vi "Experiment_CAVITY.vi"() -> ()   [LabVIEW 2009]
uses:
  <vilib>/imath/engines/lvmath2/RunTimeEngine/ErrorHandling/NIMS_Finalize Error.vi
  <vilib>/imath/engines/lvmath2/RunTimeEngine/Parser/MC_Version.vi
  <vilib>/imath/engines/lvmath2/RunTimeEngine/Managers/WorkSpace/UID Generator.vi
  <vilib>/imath/engines/lvmath2/RunTimeEngine/NodeEndStatement/NIMS_NodeEndStatement_Output.vi
  <instcachedir>/0/NIMS_NodeEndStatement_Output_B70DDD75627E4997AAE11E9955EDAA25.lvgen/NIMS_NodeEndStatement_Output_B70DDD75627E4997AAE11E9955EDAA25_001.vi
  <vilib>/imath/engines/lvmath2/RunTimeEngine/Managers/SymbolTable/Clear UID.vi
  <vilib>/imath/engines/lvmath2/RunTimeEngine/LocalVariableDefStatement/MC_LocalVariableDefStatement_Display.vi
  <vilib>/imath/engines/lvmath2/RunTimeEngine/RunTimeType/NIMS_RunTimeType_From StrictType (excl LVString).vi
  <vilib>/imath/engines/lvmath2/RunTimeEngine/RangeToken/NIMS_Range.vi
  <instcachedir>/0/NIMS_Range_6D647EC16A744C98B5DE1D649A2D648D.lvgen/NIMS_Range_6D647EC16A744C98B5DE1D649A2D648D_001.vi
  <vilib>/imath/engines/lvmath/Functions/Error Handling/error.ctl
  <vilib>/imath/engines/lvmath/Functions/Error Handling/MergeErrorsWrapper.vi
  <vilib>/imath/engines/lvmath2/RunTimeEngine/VariableToken/NIMS_VariableToken_CondDefined.vi
  <instcachedir>/0/NIMS_VariableToken_CondDefined_5641E79000FB4D628475532441475385.lvgen/NIMS_VariableToken_CondDefined_5641E79000FB4D628475532441475385_002.vi
  <vilib>/imath/engines/lvmath/Functions/Error Handling/MC_Mask_Errors.vi
  <vilib>/imath/engines/lvmath2/RunTimeEngine/BuiltInFunctions/rem/NIMS_rem_no checks.vi
  <instcachedir>/0/NIMS_rem_no checks_4CC9B305AB7E42EF90AFC4973FB32F8D.lvgen/NIMS_rem_no checks_4CC9B305AB7E42EF90AFC4973FB32F8D_000.vi
  <vilib>/imath/engines/lvmath2/RunTimeEngine/BuiltInFunctions/uint32/NIMS_uint32(real).vi
  <instcachedir>/0/NIMS_uint32(real)_FDC83D68D45943DDB8F3F934FF8A712F.lvgen/NIMS_uint32(real)_FDC83D68D45943DDB8F3F934FF8A712F_000.vi
  <vilib>/imath/engines/lvmath2/RunTimeEngine/BuiltInFunctions/double/NIMS_double.vi
  <instcachedir>/0/NIMS_double_2CE444F3CE4146B199A482FE12545E45.lvgen/NIMS_double_2CE444F3CE4146B199A482FE12545E45_000.vi
  <vilib>/imath/engines/lvmath2/RunTimeEngine/BuiltInFunctions/length/NIMS_length(GV).vi
  <instcachedir>/0/NIMS_length(GV)_7D6E94E728E145E68721C53861296D96.lvgen/NIMS_length(GV)_7D6E94E728E145E68721C53861296D96_000.vi
  <instcachedir>/0/NIMS_Range_6D647EC16A744C98B5DE1D649A2D648D.lvgen/NIMS_Range_6D647EC16A744C98B5DE1D649A2D648D_000.vi
  <vilib>/imathl/engines/lvmath/Functions/Error Handling/Create Error.vi
  <vilib>/imath/engines/lvmath2/RunTimeEngine/ReplaceToken/NIMS_Replace - V(S)=S.vi
  <instcachedir>/0/NIMS_Replace - V(S)=S_670A9E0533664C1D848C8E58B3321B6A.lvgen/NIMS_Replace - V(S)=S_670A9E0533664C1D848C8E58B3321B6A_001.vi
  <vilib>/imath/engines/lvmath2/RunTimeEngine/ReplaceToken/NIMS_Replace - Size Check _(_)=S.vi
  <instcachedir>/0/NIMS_Replace - Size Check _(_)=S_8596181D73404097BAB9CBB006194BB0.lvgen/NIMS_Replace - Size Check _(_)=S_8596181D73404097BAB9CBB006194BB0_002.vi
  <vilib>/imath/engines/lvmath2/RunTimeEngine/ReplaceToken/NIMS_Replace - Check Linear.vi
  <instcachedir>/0/NIMS_Replace - Check Linear_9243CBB174894FF6977027453DA6955E.lvgen/NIMS_Replace - Check Linear_9243CBB174894FF6977027453DA6955E_002.vi
  <vilib>/imath/engines/lvmath2/RunTimeEngine/VariableToken/NIMS_VariableToken_CondDefinedDefinedByReplace.vi
  <instcachedir>/0/NIMS_VariableToken_CondDefinedDefinedByReplace_D162CFFC24174562A9FEA619A91E1A56.lvgen/NIMS_VariableToken_CondDefinedDefinedByReplace_D162CFFC24174562A9FEA619A91E1A56_002.vi
  <vilib>/imath/engines/lvmath2/RunTimeEngine/CommandStatement/MC_CommandStatement_break.vi
  <vilib>/imath/engines/lvmath2/RunTimeEngine/ArithmeticOperatorToken/NIMS_ArithmeticOperator_times.vi
  <instcachedir>/0/NIMS_ArithmeticOperator_times_3987BC660D7947CD8628C10658A43225.lvgen/NIMS_ArithmeticOperator_times_3987BC660D7947CD8628C10658A43225_001.vi
  <instcachedir>/0/NIMS_NodeEndStatement_Output_B70DDD75627E4997AAE11E9955EDAA25.lvgen/NIMS_NodeEndStatement_Output_B70DDD75627E4997AAE11E9955EDAA25_000.vi
  <instcachedir>/0/NIMS_ArithmeticOperator_times_3987BC660D7947CD8628C10658A43225.lvgen/NIMS_ArithmeticOperator_times_3987BC660D7947CD8628C10658A43225_000.vi
  <vilib>/imath/engines/lvmath2/RunTimeEngine/VariableToken/Read/NIMS_Get Elements - RV(_) - Check.vi
  <instcachedir>/0/NIMS_Get Elements - RV(_) - Check_60F12861D0564803969A5D0D0D1716CD.lvgen/NIMS_Get Elements - RV(_) - Check_60F12861D0564803969A5D0D0D1716CD_001.vi
  <instcachedir>/0/NIMS_VariableToken_CondDefined_5641E79000FB4D628475532441475385.lvgen/NIMS_VariableToken_CondDefined_5641E79000FB4D628475532441475385_001.vi
  <instcachedir>/0/NIMS_VariableToken_CondDefined_5641E79000FB4D628475532441475385.lvgen/NIMS_VariableToken_CondDefined_5641E79000FB4D628475532441475385_003.vi
  <vilib>/imath/engines/lvmath2/RunTimeEngine/ArithmeticOperatorToken/NIMS_ArithmeticOperator_power(S).vi
  <instcachedir>/0/NIMS_ArithmeticOperator_power(S)_A502679C095F4520BDC53E297C98A9BD.lvgen/NIMS_ArithmeticOperator_power(S)_A502679C095F4520BDC53E297C98A9BD_001.vi
  <vilib>/imath/engines/lvmath2/RunTimeEngine/BuiltInFunctions/abs/NIMS_abs(signed).vi
  <instcachedir>/0/NIMS_abs(signed)_C4FCB8E6058B49B797C7C8D53CA5F6EC.lvgen/NIMS_abs(signed)_C4FCB8E6058B49B797C7C8D53CA5F6EC_000.vi
  <instcachedir>/0/NIMS_Replace - V(S)=S_670A9E0533664C1D848C8E58B3321B6A.lvgen/NIMS_Replace - V(S)=S_670A9E0533664C1D848C8E58B3321B6A_000.vi
  <instcachedir>/0/NIMS_Replace - Size Check _(_)=S_8596181D73404097BAB9CBB006194BB0.lvgen/NIMS_Replace - Size Check _(_)=S_8596181D73404097BAB9CBB006194BB0_001.vi
  <instcachedir>/0/NIMS_Replace - Check Linear_9243CBB174894FF6977027453DA6955E.lvgen/NIMS_Replace - Check Linear_9243CBB174894FF6977027453DA6955E_001.vi
  <instcachedir>/0/NIMS_VariableToken_CondDefinedDefinedByReplace_D162CFFC24174562A9FEA619A91E1A56.lvgen/NIMS_VariableToken_CondDefinedDefinedByReplace_D162CFFC24174562A9FEA619A91E1A56_001.vi
  <instcachedir>/0/NIMS_Replace - V(S)=S_670A9E0533664C1D848C8E58B3321B6A.lvgen/NIMS_Replace - V(S)=S_670A9E0533664C1D848C8E58B3321B6A_002.vi
  <instcachedir>/0/NIMS_Replace - Size Check _(_)=S_8596181D73404097BAB9CBB006194BB0.lvgen/NIMS_Replace - Size Check _(_)=S_8596181D73404097BAB9CBB006194BB0_003.vi
  <instcachedir>/0/NIMS_Replace - Check Linear_9243CBB174894FF6977027453DA6955E.lvgen/NIMS_Replace - Check Linear_9243CBB174894FF6977027453DA6955E_003.vi
  <instcachedir>/0/NIMS_VariableToken_CondDefinedDefinedByReplace_D162CFFC24174562A9FEA619A91E1A56.lvgen/NIMS_VariableToken_CondDefinedDefinedByReplace_D162CFFC24174562A9FEA619A91E1A56_003.vi
  <instcachedir>/0/NIMS_abs(signed)_C4FCB8E6058B49B797C7C8D53CA5F6EC.lvgen/NIMS_abs(signed)_C4FCB8E6058B49B797C7C8D53CA5F6EC_001.vi
  <instcachedir>/0/NIMS_NodeEndStatement_Output_B70DDD75627E4997AAE11E9955EDAA25.lvgen/NIMS_NodeEndStatement_Output_B70DDD75627E4997AAE11E9955EDAA25_003.vi
  <vilib>/imath/engines/lvmath2/RunTimeEngine/Managers/SymbolTable/NIMS_WorkSpace.lvlib
panel:
  out "error out":errorcluster
  out "error out":errorcluster
  out "error out":errorcluster
  out "error out":errorcluster
  in  "?":enum32{"CAVITY"}(tab)
  in  "FIRST 3dB POINT":bool
  in  "?":dbl(slide) scale=8.0..12.5 scale format="%#.6g"
  out "Qdesigned":dbl
  in  "RESONANT FREQUENCY":dbl(slide) scale=8.5..12.0
  out "?":errorcluster
  out "?":cluster{"Y":dbl[], "Y":dbl[]}[](graph)
  out "frequency":dbl
  out "power(dB)":cdb
  in  "SECOND 3dB POINT":bool
  in  "BAND WIDTH":bool
  in  "Q FACTOR":bool
  in  "POWER(dB) at RESONANCE":bool
  out "?":dbl
  out "?":dbl
  out "?":dbl
  out "?":dbl
  out "?":dbl
  in  "HELP FOR CAVITY":bool
  in  "?":enum32{"ATTENUATOR"}(tab)
  out "?":dbl[](graph)
  in  "Set the value of attenuation in dB":dbl(slide) scale=0.0..10.0
  out "?":errorcluster
  in  "HELP FOR ATTENUATOR":bool
  out "error out":errorcluster
  in  "?":enum32{"ISOLATOR"}(tab)
  out "?":dbl[](graph)
  in  "?":bool
  out "?":errorcluster
  in  "HELP FOR ISOLATOR":bool
  in  "?":enum32{"MODULATOR"}(tab)
  out "?":dbl[](graph)
  in  "Modulating Frequency(KHz)":dbl(slide) scale=0.5..1.5
  out "?":errorcluster
  in  "HELP FOR MODULATOR":bool
  in  "?":enum32{"SOURCE"}(tab)
  out "?":dbl[](graph)
  in  "Frequency of carrier wave(GHz)":dbl(slide) scale=8.2..12.4
  in  "Voltage":dbl(knob) scale=0.0..20.0 scale format="%#_10g"
  out "?":errorcluster
  in  "HELP FOR SOURCE":bool
  # "VSWR Meter"
  # "Source"
  # "Variable Attenuator"
  # "Cavity"
  # "Coaxial to rectangular adapter"
  # "Isolator"
  # "Connecting waveguide"
  # "Connecting waveguide"
  # "Matched load"
  # "Backward Direction"
  # "Forward direction"
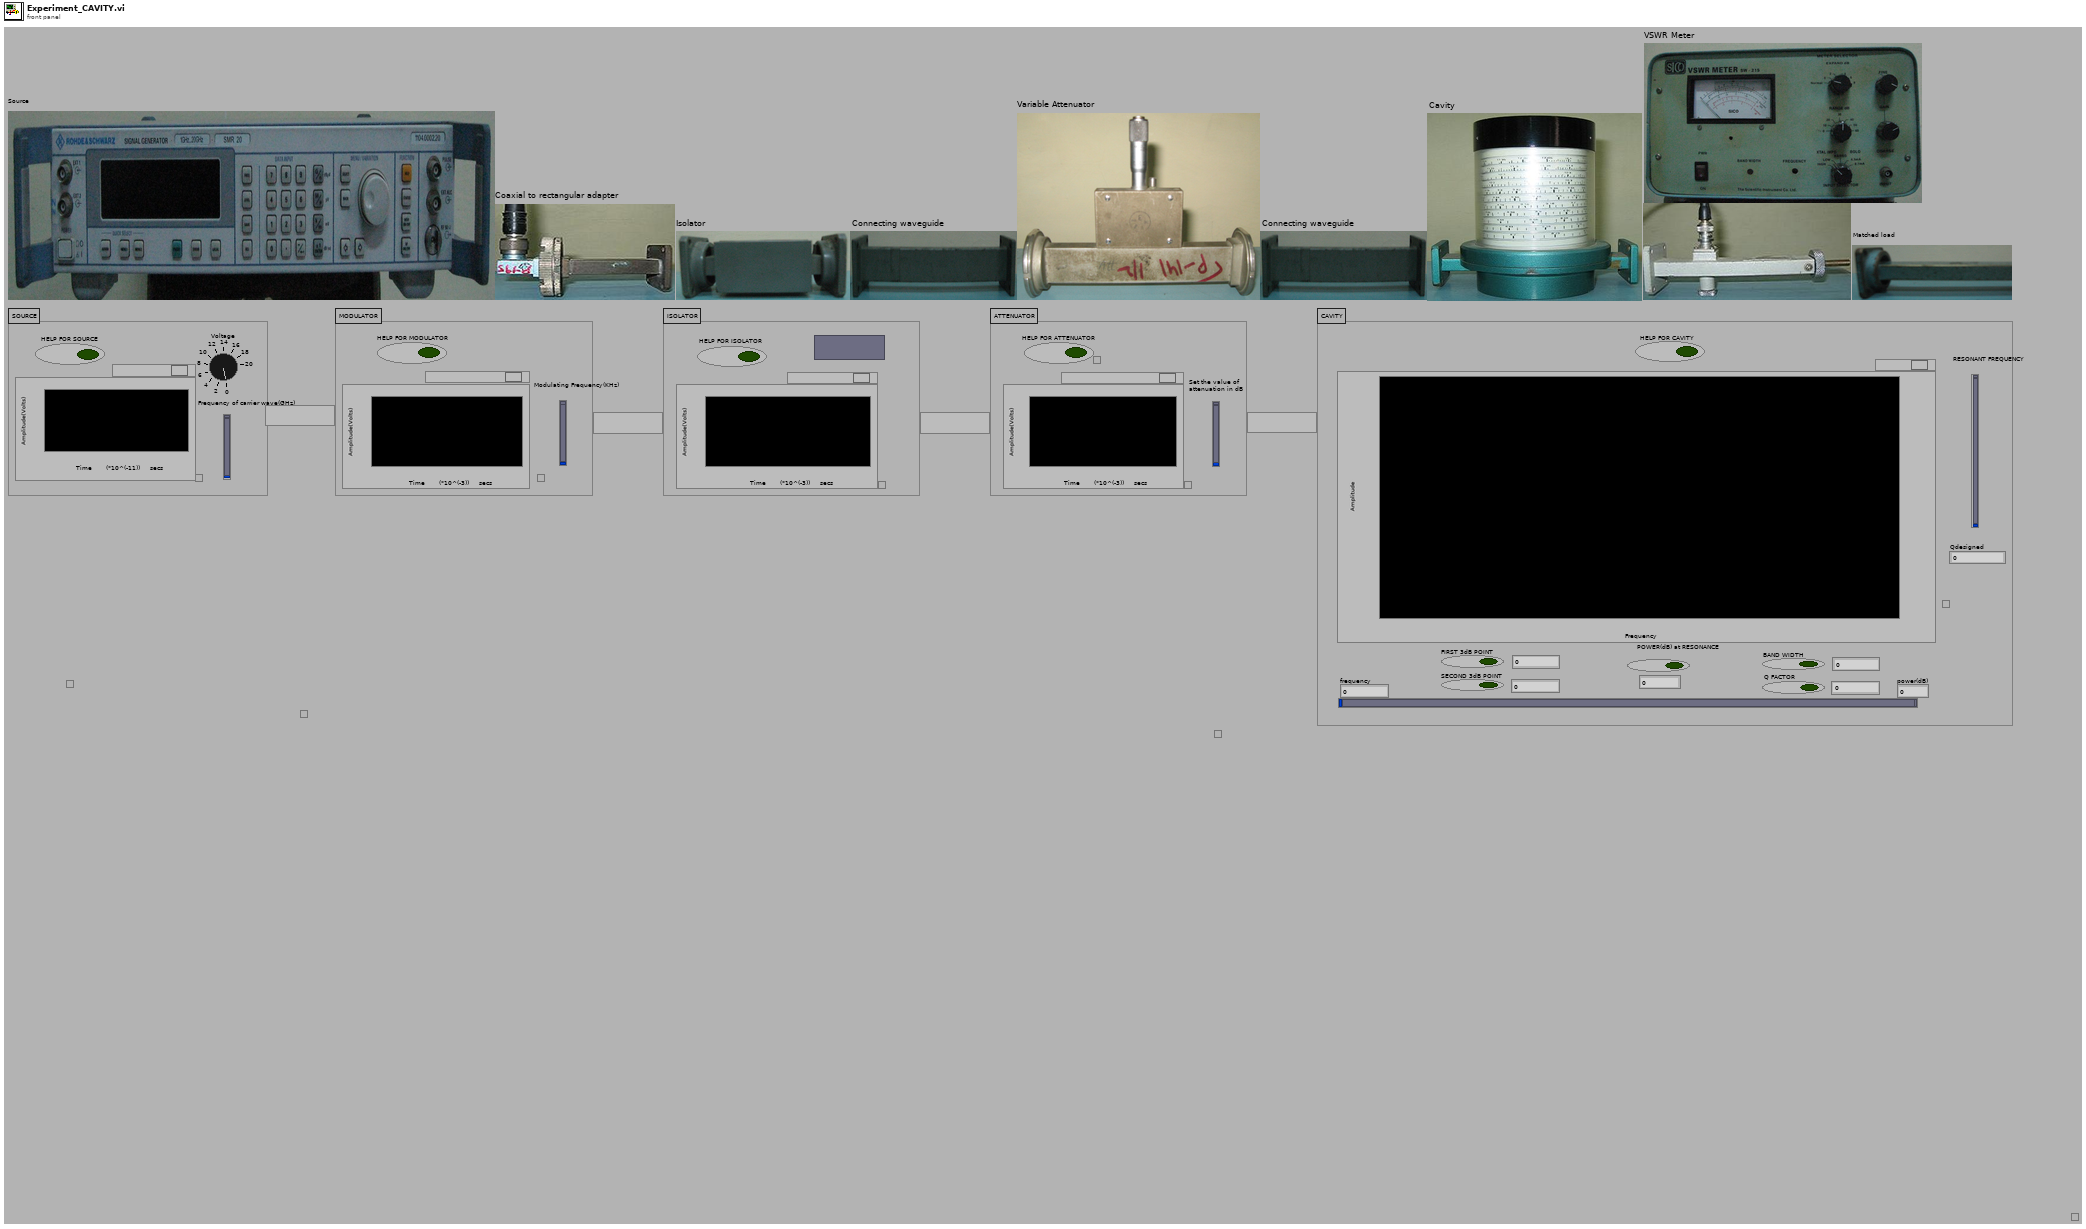
[diagram p1: front panel]
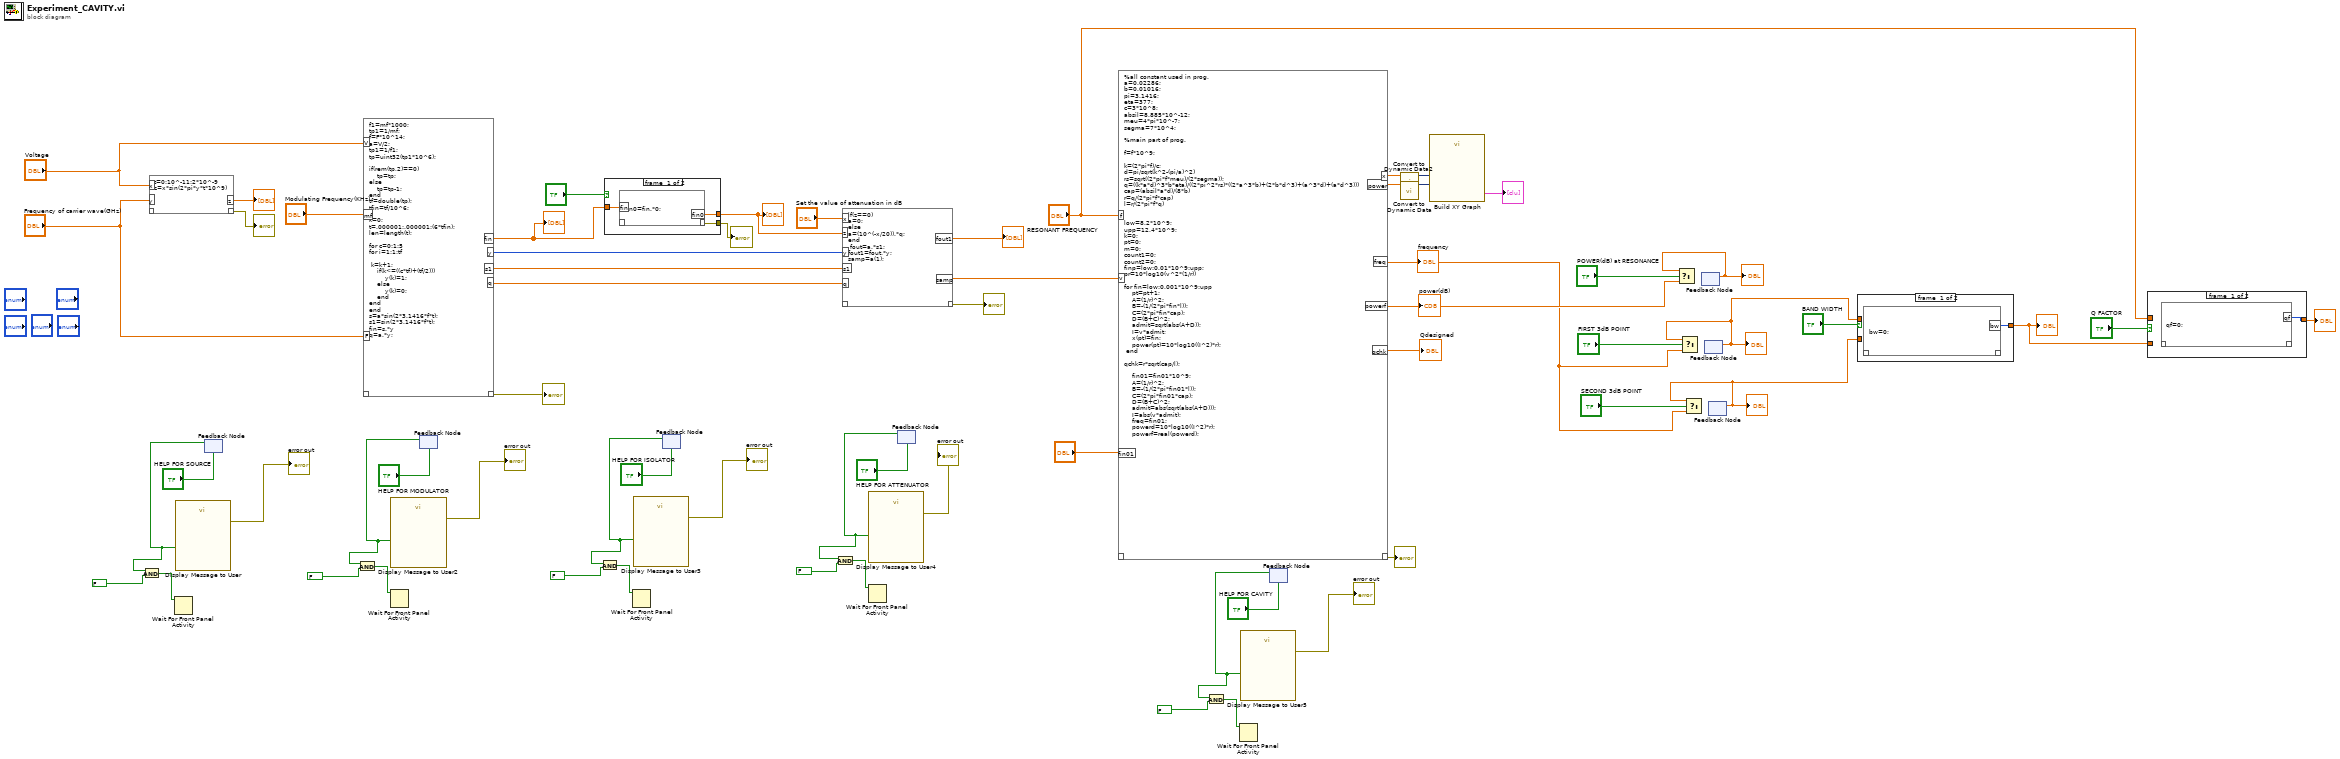
[diagram p0: block diagram]
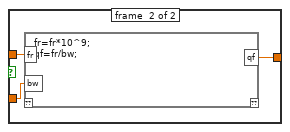
[diagram p2: hidden frame]
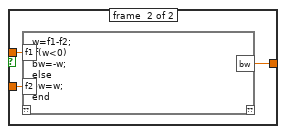
[diagram p3: hidden frame]
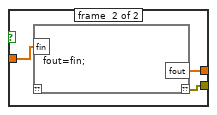
[diagram p4: hidden frame]
diagram:
  n1 = mathscript code="t=0:10^-11:2*10^-9\nz=x*sin(2*pi*y*t*10^9)"("x"="Voltage", "y"="Frequency of carrier wave(GHz)") -> ("??"=→"?":errorcluster, "z"=→"?":dbl[])  [unwired: 1 in]
  n2 = feedback #1("HELP FOR SOURCE") -> (w27:bool)
  n3 = And(x=w27, y=FALSE) -> (x .and. y?=w25:bool)
  n4 = Wait For Front Panel Activity(3:w25) -> ()  [unwired: 3 out]
  n5 = call "Display Message to User"("Enable"=w27) -> ("error out"=→"error out":errorcluster, "CLOSE"=w29:bool)  [unwired: 2 in, 7 out]
  n6 = mathscript code="f1=mf*1000;\ntp1=1/mf;\nf=F*10^14;\na=V/2;\ntp1=1/f1;\ntp=uint32(tp1*10^6);\n\nif(rem(tp,2)==0)\n    tp=tp;\nelse\n    tp=tp-1;\nend\ntf=double(tp);\ntfin=tf/10^6;\n\nk=0;\nt=.000001:.000001:(6*tfin);\nlen=length(t);\n\nfor c=0:1:5\nfor i=1:1:tf\n  \n k=k+1;\n    if(k<=((c*tf)+(tf/2)))\n        y(k)=1;\n    else\n        y(k)=0;\n    end\nend\nend\ns=a*sin(2*3.1416*f*t);\ns1=sin(2*3.1416*f*t);\nfin=s.*y\nq=a.*y;"("V"="Voltage", "mf"="Modulating Frequency(KHz)", "F"="Frequency of carrier wave(GHz)") -> ("??"=→"?":errorcluster, "y"=w57:i32[], "q"=w55:dbl[], "fin"=w62:dbl[], "s1"=w56:dbl[])  [unwired: 1 in]
  "?" <- w62
  n7 = feedback #2("HELP FOR MODULATOR") -> (w21:bool)
  n8 = And(x=w21, y=FALSE) -> (x .and. y?=w19:bool)
  n9 = Wait For Front Panel Activity(3:w19) -> ()  [unwired: 3 out]
  n10 = call "Display Message to User2"("Enable"=w21) -> ("error out"=→"error out":errorcluster, "CLOSE"=w23:bool)  [unwired: 2 in, 7 out]
  n11 = case shown="False" "?" {
    tunnel: [w73 w94] -> w58
    tunnel: w62 -> [w74 w95]
    tunnel: [w72 w93] -> w60
    frame #0 {
      n12 = mathscript code="fin0=fin.*0;"("fin"=w74) -> ("??"=w72:errorcluster, "fin0"=w73:dbl[])  [unwired: 1 in]
    }
    frame #1 {
      n13 = mathscript code="fout=fin;"("fin"=w95) -> ("??"=w93:errorcluster, "fout"=w94:dbl[])  [unwired: 1 in]
    }
  }
  "?" <- w58
  "?" <- w60
  n14 = feedback #3("HELP FOR ISOLATOR") -> (w15:bool)
  n15 = And(x=w15, y=FALSE) -> (x .and. y?=w13:bool)
  n16 = Wait For Front Panel Activity(3:w13) -> ()  [unwired: 3 out]
  n17 = call "Display Message to User3"("Enable"=w15) -> ("error out"=→"error out":errorcluster, "CLOSE"=w17:bool)  [unwired: 2 in, 7 out]
  n18 = mathscript code="if(z==0)\na=0; \nelse\na=(10^(-x/20)).*q;\nend\n fout=a.*s1;\nfout1=fout.*y;\nsamp=a(1);"("x"="Set the value of attenuation in dB", "z"=w58, "y"=w57, "s1"=w56, "q"=w55) -> ("??"=→"?":errorcluster, "fout1"=→"?":dbl[], "samp"=w67:dbl)  [unwired: 1 in]
  n19 = feedback #4("HELP FOR ATTENUATOR") -> (w9:bool)
  n20 = And(x=w9, y=FALSE) -> (x .and. y?=w7:bool)
  n21 = Wait For Front Panel Activity(3:w7) -> ()  [unwired: 3 out]
  n22 = call "Display Message to User4"("Enable"=w9) -> ("error out"=→"error out":errorcluster, "CLOSE"=w11:bool)  [unwired: 2 in, 7 out]
  n23 = mathscript code="%all constant used in prog.\na=0.02286;\nb=0.01016;\npi=3.1416;\neta=377;\nc=3*10^8;\nabsil=8.885*10^-12;\nmeu=4*pi*10^-7;\nsegma=7*10^4;\n\n%main part of prog.\n\nf=f*10^9;\n\nk=(2*pi*f)/c;\nd=pi/sqrt(k^2-(pi/a)^2)\nrs=sqrt((2*pi*f*meu)/(2*segma));\nq=((k*a*d)^3*b*eta)/((2*pi^2*rs)*((2*a^3*b)+(2*b*d^3)+(a^3*d)+(a*d^3)))\ncap=(absil*a*d)/(8*b)\nr=q/(2*pi*f*cap)\nl=r/(2*pi*f*q)\n\n\nlow=8.2*10^9;\nupp=12.4*10^9;\nk=0;\npt=0;\nm=0;\ncount1=0;\ncount2=0;\nfinp=low:0.01*10^9:upp;\npr=10*log10(v^2*(1/r))\n\nfor fin=low:0.001*10^9:upp\n    pt=pt+1;\n    A=(1/r)^2;\n    B=-(1/(2*pi*fin*l));\n    C=(2*pi*fin*cap);\n    D=(B+C)^2;\n    admit=sqrt(abs(A+D));\n    I=v*admit;\n    x(pt)=fin;\n    power(pt)=10*log10((I^2)*r);\n end\n\nqchk=r*sqrt(cap/l);\n    \n    fin01=fin01*10^9;\n    A=(1/r)^2;\n    B=-(1/(2*pi*fin01*l));\n    C=(2*pi*fin01*cap);\n    D=(B+C)^2;\n    admit=abs(sqrt(abs(A+D)));\n    I=abs(v*admit);\n    freq=fin01;\n    powerd=10*log10((I^2)*r);\n    powerf=real(powerd);"("v"=w67, "f"="RESONANT FREQUENCY", "fin01"="?") -> ("??"=→"?":errorcluster, "power"=w51:dbl[], "qchk"=→"Qdesigned":dbl, "x"=w49:dbl[], "freq"=w39:dbl, "powerf"=w44:dbl)  [unwired: 1 out]
  "frequency" <- w39
  "power(dB)" <- w44
  n24 = feedback #5("HELP FOR CAVITY") -> (w3:bool)
  n25 = And(x=w3, y=FALSE) -> (x .and. y?=w1:bool)
  n26 = Wait For Front Panel Activity(3:w1) -> ()  [unwired: 3 out]
  n27 = call "Display Message to User5"("Enable"=w3) -> ("error out"=→"error out":errorcluster, "CLOSE"=w5:bool)  [unwired: 2 in, 7 out]
  n28 = call "Convert to Dynamic Data2"("Array"=w49) -> ("Dynamic Data Type"=w48:dynamicdata)  [unwired: 3 in]
  n29 = call "Convert to Dynamic Data"("Array"=w51) -> ("Dynamic Data Type"=w50:dynamicdata)  [unwired: 3 in]
  n30 = call "Build XY Graph"("Y Input"=w50, "X Input"=w48) -> ("XY Graph"=→"?":cluster{"Y":dbl[], "Y":dbl[]}[])  [unwired: 8 in, 1 out]
  n31 = feedback #6() -> (w37:dbl)  [unwired: 1 in]
  "?" <- w37
  n32 = Select(t=w37, s="POWER(dB) at RESONANCE", f=w44) -> (s? t:f=w46:dbl)
  n33 = feedback #7() -> (w32:dbl)  [unwired: 1 in]
  "?" <- w32
  n34 = Select(t=w32, s="FIRST 3dB POINT", f=w39) -> (s? t:f=w43:dbl)
  n35 = feedback #8() -> (w31:dbl)  [unwired: 1 in]
  "?" <- w31
  n36 = Select(t=w31, s="SECOND 3dB POINT", f=w39) -> (s? t:f=w41:dbl)
  n37 = case shown="True" "BAND WIDTH" {
    tunnel: w31 -> [_ w129]
    tunnel: [w112 w128] -> w34
    tunnel: w32 -> [_ w127]
    frame #0 {
      n38 = mathscript code="bw=0;"() -> ("bw"=w112:i32)  [unwired: 1 in, 1 out]
    }
    frame #1 {
      n39 = mathscript code="w=f1-f2;\nif(w<0)\nbw=-w;\nelse\nbw=w;\nend"("f1"=w127, "f2"=w129) -> ("bw"=w128:dbl)  [unwired: 1 in, 1 out]
    }
  }
  "?" <- w34
  n40 = case shown="True" "Q FACTOR" {
    tunnel: "RESONANT FREQUENCY" -> [_ w187]
    tunnel: w34 -> [_ w186]
    tunnel: [w170 w185] -> w33
    frame #0 {
      n41 = mathscript code="qf=0;"() -> ("qf"=w170:i32)  [unwired: 1 in, 1 out]
    }
    frame #1 {
      n42 = mathscript code="fr=fr*10^9;\nqf=fr/bw;"("fr"=w187, "bw"=w186) -> ("qf"=w185:dbl)  [unwired: 1 in, 1 out]
    }
  }
  "?" <- w33
